vi "Dresden R2R Sputter 03.02.2018 IY24.vi"() -> ()   [LabVIEW 2009] (continued)
                                n28534 = case shown="False" w33549 {
                                frame #0 {
                                n28535 = local read "R Set Pressure mtorr"() -> (w33554:dbl)
                                n28536 = local write "Set_pressure_value 4"(w33554) -> ()
                                }
                                frame #1 {
                                }
                                }
                                }
                                frame #1 {
                                }
                                }
                                }
                                frame #5 {
                                n28537 = local read "Semi"() -> (w33555:bool)
                                n28538 = case shown="False" w33555 {
                                frame #0 {
                                n28539 = local read "Set_pressure_value 4"() -> (w33557:dbl)
                                n28540 = Add(x=1.0, y=w33557) -> (x+y=w33559:dbl)
                                n28541 = Subtract(x=w33557, y=1.0) -> (x-y=w33560:dbl)
                                n28542 = local read "Pressure 4"() -> (w33556:i32)
                                n28543 = In Range and Coerce(upper limit=w33559, x=w33556, lower limit=w33560) -> (In Range?=w33558:bool)  [unwired: 1 out]
                                n28544 = case shown="False" w33558 {
                                frame #0 {
                                n28545 = local write "Pc_bv4_auto_set_pressure"(TRUE ("Pc_bv1_auto_set_pressure")) -> ()
                                }
                                frame #1 {
                                }
                                }
                                }
                                frame #1 {
                                }
                                }
                                }
                                frame #6 {
                                n28546 = local read "Semi"() -> (w33564:bool)
                                n28547 = case shown="False" w33564 {
                                frame #0 {
                                n28548 = while {
                                i -> [w33575]
                                stop <- w33567 stop-if-true
                                n28549 = Greater?(x=w33575, y=300) -> (0:w33569:bool)
                                n28550 = local read "Set_pressure_value 4"() -> (w33566:dbl)
                                n28551 = Add(x=1.0, y=w33566) -> (x+y=w33571:dbl)
                                n28552 = Subtract(x=w33566, y=1.0) -> (x-y=w33572:dbl)
                                n28553 = local read "Pressure 4"() -> (w33565:i32)
                                n28554 = In Range and Coerce(upper limit=w33571, x=w33565, lower limit=w33572) -> (In Range?=w33570:bool)  [unwired: 1 out]
                                n28555 = case shown="False" w33570 {
                                tunnel: [FALSE TRUE] -> w33568
                                frame #0 {
                                n28556 = Wait Until Next ms Multiple(millisecond multiple=u32 200) -> ()  [unwired: 1 out]
                                }
                                frame #1 {
                                }
                                }
                                n28557 = Or(x=w33568, y=w33569) -> (x .or. y?=w33567:bool)
                                }
                                }
                                frame #1 {
                                }
                                }
                                }
                                frame #7 {
                                n28558 = local read "Semi"() -> (w33580:bool)
                                n28559 = case shown="False" w33580 {
                                frame #0 {
                                n28560 = local read "Set_pressure_value 4"() -> (w33582:dbl)
                                n28561 = Add(x=1.0, y=w33582) -> (x+y=w33584:dbl)
                                n28562 = Subtract(x=w33582, y=1.0) -> (x-y=w33585:dbl)
                                n28563 = local read "Pressure 4"() -> (w33581:i32)
                                n28564 = In Range and Coerce(upper limit=w33584, x=w33581, lower limit=w33585) -> (In Range?=w33583:bool)  [unwired: 1 out]
                                n28565 = case shown="False" w33583 {
                                frame #0 {
                                n28566 = local write "Semi"(TRUE ("Semi")) -> ()
                                n28567 = local write "Error Message"("Coating Pressure could not be adjusted !" ("Error Message")) -> ()
                                }
                                frame #1 {
                                }
                                }
                                }
                                frame #1 {
                                }
                                }
                                }
                                }
                                }
                                frame #1 {
                                }
                                }
                                }
                                frame #1 {
                                n28568 = local read "Semi"() -> (w33590:bool)
                                n28569 = case shown="False" w33590 {
                                frame #0 {
                                n28570 = local write "SDC1 9"(TRUE ("SDC1 9")) -> ()
                                n28571 = Wait (ms)(milliseconds to wait=u32 1000) -> ()  [unwired: 1 out]
                                }
                                frame #1 {
                                }
                                }
                                }
                                }
                                }
                                }
                                }
                                frame #15 {
                                # "DC -Ignite Plasma"
                                n28572 = stacked-sequence {
                                frame #0 {
                                n28573 = local read "Semi"() -> (w33593:bool)
                                n28574 = case shown="False" w33593 {
                                frame #0 {
                                n28575 = stacked-sequence {
                                frame #0 {
                                n28576 = local read "Semi"() -> (w33594:bool)
                                n28577 = case shown="False" w33594 {
                                frame #0 {
                                n28578 = local write "RF_host_auto"(TRUE ("Dc_host_auto")) -> ()
                                }
                                frame #1 {
                                }
                                }
                                }
                                frame #1 {
                                n28579 = local read "Semi"() -> (w33596:bool)
                                n28580 = case shown="False" w33596 {
                                frame #0 {
                                n28581 = local read "R Single RF  Step1 Coating Power"() -> (w33597:dbl)
                                n28582 = local write "RF_forward_power_1"(w33597) -> ()
                                }
                                frame #1 {
                                }
                                }
                                }
                                frame #2 {
                                n28583 = local read "Semi"() -> (w33598:bool)
                                n28584 = case shown="False" w33598 {
                                frame #0 {
                                n28585 = Wait (ms)(milliseconds to wait=u32 1000) -> ()  [unwired: 1 out]
                                }
                                frame #1 {
                                }
                                }
                                }
                                frame #3 {
                                n28586 = local read "Semi"() -> (w33600:bool)
                                n28587 = case shown="False" w33600 {
                                frame #0 {
                                n28588 = local write "RF set auto"(TRUE ("Dc_auto_set")) -> ()
                                }
                                frame #1 {
                                }
                                }
                                }
                                frame #4 {
                                n28589 = Wait (ms)(milliseconds to wait=u32 1000) -> ()  [unwired: 1 out]
                                }
                                frame #5 {
                                n28590 = local read "Semi"() -> (w33603:bool)
                                n28591 = case shown="False" w33603 {
                                frame #0 {
                                n28592 = local read "Web_selection_tab"() -> (w33604:T5)
                                n28593 = case shown="\"Other                                                                                    \"" w33604 {
                                frame #0 {
                                }
                                frame #1 {
                                n28594 = local write "RF_auto_on"(TRUE ("Dc_auto_on")) -> ()
                                }
                                }
                                }
                                frame #1 {
                                }
                                }
                                }
                                frame #6 {
                                n28595 = local read "Web_selection_tab"() -> (w33606:T5)
                                n28596 = case shown="\"Other                                                                                    \"" w33606 {
                                frame #0 {
                                }
                                frame #1 {
                                n28597 = local read "Semi"() -> (w33607:bool)
                                n28598 = case shown="False" w33607 {
                                frame #0 {
                                n28599 = while {
                                i -> [w33617]
                                stop <- w33610 stop-if-true
                                n28600 = Greater Or Equal?(x=w33617, y=240) -> (x >= y?=w33616:bool)
                                n28601 = case shown="True" w33616 {
                                frame #0 {
                                }
                                frame #1 {
                                n28602 = local write "Semi"(TRUE ("Semi")) -> ()
                                }
                                }
                                n28603 = local read "RF_forward_power_1"() -> (w33608:i16)
                                n28604 = local read "RF Net Power :"() -> (w33609:u32)
                                n28605 = Subtract(x=w33608, y=w33609) -> (x-y=w33615:u32)
                                n28606 = Less?(x=w33615, y=10.0) -> (x < y?=w33612:bool)
                                n28607 = local read "Semi"() -> (w33611:bool)
                                n28608 = Or(x=w33612, y=w33611) -> (x .or. y?=w33610:bool)
                                n28609 = Wait Until Next ms Multiple(millisecond multiple=u32 500) -> ()  [unwired: 1 out]
                                }
                                }
                                frame #1 {
                                }
                                }
                                }
                                }
                                }
                                frame #7 {
                                n28610 = local read "Semi"() -> (w33620:bool)
                                n28611 = case shown="False" w33620 {
                                frame #0 {
                                n28612 = Wait (ms)(milliseconds to wait=u32 1000) -> ()  [unwired: 1 out]
                                }
                                frame #1 {
                                }
                                }
                                }
                                }
                                }
                                frame #1 {
                                }
                                }
                                }
                                frame #1 {
                                n28613 = local read "Semi"() -> (w33622:bool)
                                n28614 = case shown="False" w33622 {
                                frame #0 {
                                n28615 = Wait (ms)(milliseconds to wait=u32 1000) -> ()  [unwired: 1 out]
                                n28616 = local write "SDC1 13"(TRUE ("SDC1 13")) -> ()
                                }
                                frame #1 {
                                }
                                }
                                }
                                }
                                }
                                frame #16 {
                                n28617 = local read "Web_selection_tab"() -> (w33625:T5)
                                n28618 = case shown="\"Web                                                                                    \", Default" w33625 {
                                frame #0 {
                                n28619 = stacked-sequence {
                                frame #0 {
                                n28620 = local read "R Minimum diameter"() -> (w33626:dbl)
                                n28621 = local read "R Maximum diameter"() -> (w33627:dbl)
                                n28622 = local read "R Web thicness"() -> (w33628:dbl)
                                n28623 = local read "R Web speed(cm/min)"() -> (w33629:dbl)
                                n28624 = Wait (ms)(milliseconds to wait=u32 100) -> ()  [unwired: 1 out]
                                n28625 = local write "Initial Min Diameter"(w33626) -> ()
                                n28626 = local write "Max Diameter"(w33627) -> ()
                                n28627 = local write "Web Thickness"(w33628) -> ()
                                n28628 = local write "Web Speed"(w33629) -> ()
                                }
                                frame #1 {
                                n28629 = local read "R Single RF Step1 Coating Power Active"() -> (w33644:bool)
                                n28630 = local read "R Single RF Step2 Coating Power Active"() -> (w33643:bool)
                                n28631 = local read "R Single RF Step3 Coating Power Active"() -> (w33642:bool)
                                n28632 = local read "R Single RF Step4 Coating Power Active"() -> (w33641:bool)
                                n28633 = local read "R Single RF Step5 Coating Power Active"() -> (w33640:bool)
                                n28634 = Boolean To (0,1)(Boolean=w33644) -> (0, 1=w33639:i16)
                                n28635 = Boolean To (0,1)(Boolean=w33643) -> (0, 1=w33638:i16)
                                n28636 = Boolean To (0,1)(Boolean=w33642) -> (0, 1=w33637:i16)
                                n28637 = Boolean To (0,1)(Boolean=w33641) -> (0, 1=w33636:i16)
                                n28638 = Boolean To (0,1)(Boolean=w33640) -> (0, 1=w33635:i16)
                                n28639 = Compound Arithmetic op=ADD(w33639, w33638, w33637, w33636, w33635) -> (w33633:i16)
                                n28640 = local read "R Single RF Interval length"() -> (w33634:dbl)
                                n28641 = Wait (ms)(milliseconds to wait=u32 200) -> ()  [unwired: 1 out]
                                n28642 = Multiply(x=w33634, y=w33633) -> (x*y=w33632:dbl)
                                n28643 = local write "Total length"(w33632) -> ()
                                }
                                frame #2 {
                                n28644 = local write "Calculate 2"(TRUE ("Calculate_auto")) -> ()
                                n28645 = Wait (ms)(milliseconds to wait=u32 200) -> ()  [unwired: 1 out]
                                }
                                frame #3 {
                                n28646 = local write "Roll_side_select"(enum32{"Left to Right", "Right to Left"}."Left to Right" ("Roll_side_select")) -> ()
                                n28647 = Wait (ms)(milliseconds to wait=u32 200) -> ()  [unwired: 1 out]
                                }
                                frame #4 {
                                n28648 = Wait (ms)(milliseconds to wait=u32 100) -> ()  [unwired: 1 out]
                                n28649 = local write "Parameters_auto_set"(TRUE ("Parameters_auto_set")) -> ()
                                }
                                frame #5 {
                                n28650 = while {
                                i -> [w33655]
                                stop <- w33651 stop-if-true
                                n28651 = Wait Until Next ms Multiple(millisecond multiple=u32 300) -> ()  [unwired: 1 out]
                                n28652 = Greater?(x=w33655, y=100) -> (0:w33652:bool)
                                n28653 = local read "Parameters_auto_set"() -> (w33656:bool)
                                n28654 = case shown="False" w33656 {
                                tunnel: [TRUE FALSE] -> w33653
                                frame #0 {
                                }
                                frame #1 {
                                }
                                }
                                n28655 = Or(x=w33653, y=w33652) -> (x .or. y?=w33651:bool)
                                }
                                }
                                frame #6 {
                                n28656 = local read "R Tension Value"() -> (w33660:dbl)
                                n28657 = Wait (ms)(milliseconds to wait=u32 200) -> ()  [unwired: 1 out]
                                n28658 = local write "TC1_set_value"(w33660) -> ()
                                }
                                frame #7 {
                                n28659 = local write "TC1_auto_set"(TRUE ("TC1_auto_set")) -> ()
                                }
                                frame #8 {
                                w33664 = u16 3 items=["1", "2", "3", "4"] ("Target Chamber Sensor")
                                n28660 = local write "Target Chamber Sensor"(w33664) -> ()
                                n28661 = Wait (ms)(milliseconds to wait=u32 200) -> ()  [unwired: 1 out]
                                }
                                frame #9 {
                                n28662 = local read "Total length"() -> (w33665:dbl)
                                n28663 = local write "Region"(w33665) -> ()
                                }
                                frame #10 {
                                n28664 = local read "Semi"() -> (w33666:bool)
                                n28665 = case shown="False" w33666 {
                                frame #0 {
                                n28666 = stacked-sequence {
                                frame #0 {
                                # "Gas Flow"
                                n28667 = stacked-sequence {
                                frame #0 {
                                n28668 = local read "Semi"() -> (w33667:bool)
                                n28669 = case shown="False" w33667 {
                                frame #0 {
                                n28670 = stacked-sequence {
                                frame #0 {
                                n28671 = local read "Semi"() -> (w33668:bool)
                                n28672 = case shown="False" w33668 {
                                frame #0 {
                                n28673 = local read "R Argon Flow sccm"() -> (w33669:dbl)
                                n28674 = local write "Ar_sccm3_4"(w33669) -> ()
                                }
                                frame #1 {
                                }
                                }
                                }
                                frame #1 {
                                n28675 = local read "Semi"() -> (w33670:bool)
                                n28676 = case shown="False" w33670 {
                                frame #0 {
                                n28677 = local write "Mfc2_Ar _3_4_set"(TRUE ("Mfc_Ar _1_2_set")) -> ()
                                }
                                frame #1 {
                                }
                                }
                                }
                                frame #2 {
                                n28678 = local read "Semi"() -> (w33672:bool)
                                n28679 = case shown="False" w33672 {
                                frame #0 {
                                n28680 = while {
                                i -> [w33675]
                                stop <- w33677 stop-if-true
                                n28681 = Greater?(x=w33675, y=50) -> (0:w33674:bool)
                                n28682 = local read "Semi"() -> (w33673:bool)
                                n28683 = Or(x=w33673, y=w33674) -> (x .or. y?=w33677:bool)
                                }
                                }
                                frame #1 {
                                }
                                }
                                }
                                frame #3 {
                                n28684 = local read "Semi"() -> (w33678:bool)
                                n28685 = case shown="False" w33678 {
                                frame #0 {
                                n28686 = local read "Ar_sccm_act 2"() -> (w33679:dbl)
                                n28687 = Greater?(x=w33679, y=1) -> (0:w33680:bool)
                                n28688 = case shown="False" w33680 {
                                frame #0 {
                                n28689 = local read "R Argon Flow sccm"() -> (w33682:dbl)
                                n28690 = local write "Ar_sccm3_4"(w33682) -> ()
                                }
                                frame #1 {
                                }
                                }
                                }
                                frame #1 {
                                }
                                }
                                }
                                frame #4 {
                                n28691 = local read "Semi"() -> (w33683:bool)
                                n28692 = case shown="False" w33683 {
                                frame #0 {
                                n28693 = local read "Ar_sccm_act 2"() -> (w33684:dbl)
                                n28694 = Greater?(x=w33684, y=1) -> (0:w33685:bool)
                                n28695 = case shown="False" w33685 {
                                frame #0 {
                                n28696 = while {
                                i -> [w33688]
                                stop <- w33692 stop-if-true
                                n28697 = Greater?(x=w33688, y=50) -> (0:w33687:bool)
                                n28698 = local read "Semi"() -> (w33691:bool)
                                n28699 = case shown="False" w33691 {
                                tunnel: [FALSE TRUE] -> w33690
                                frame #0 {
                                n28700 = Wait Until Next ms Multiple(millisecond multiple=u32 200) -> ()  [unwired: 1 out]
                                }
                                frame #1 {
                                }
                                }
                                n28701 = Or(x=w33690, y=w33687) -> (x .or. y?=w33692:bool)
                                }
                                }
                                frame #1 {
                                }
                                }
                                }
                                frame #1 {
                                }
                                }
                                }
                                frame #5 {
                                n28702 = local read "Semi"() -> (w33696:bool)
                                n28703 = case shown="False" w33696 {
                                frame #0 {
                                n28704 = local read "Ar_sccm_act 2"() -> (w33697:dbl)
                                n28705 = Greater?(x=w33697, y=1) -> (0:w33698:bool)
                                n28706 = case shown="False" w33698 {
                                frame #0 {
                                n28707 = local write "Semi"(TRUE ("Semi")) -> ()
                                n28708 = local write "Error Message"("Coating process cancelled.\nPlease check connections." ("Error Message")) -> ()
                                }
                                frame #1 {
                                }
                                }
                                }
                                frame #1 {
                                }
                                }
                                }
                                }
                                }
                                frame #1 {
                                }
                                }
                                }
                                frame #1 {
                                n28709 = local read "Semi"() -> (w33702:bool)
                                n28710 = case shown="False" w33702 {
                                frame #0 {
                                n28711 = local write "SDC1 11"(TRUE ("SDC1 11")) -> ()
                                n28712 = Wait (ms)(milliseconds to wait=u32 1000) -> ()  [unwired: 1 out]
                                }
                                frame #1 {
                                }
                                }
                                }
                                }
                                }
                                frame #1 {
                                # "Set Pressure for ignite plasma"
                                n28713 = stacked-sequence {
                                frame #0 {
                                n28714 = local read "Semi"() -> (w33705:bool)
                                n28715 = case shown="False" w33705 {
                                frame #0 {
                                n28716 = stacked-sequence {
                                frame #0 {
                                n28717 = local read "Semi"() -> (w33706:bool)
                                n28718 = case shown="False" w33706 {
                                frame #0 {
                                n28719 = local write "Set_pressure_value 4"(10.0 ("Set_pressure_value 2")) -> ()
                                }
                                frame #1 {
                                }
                                }
                                }
                                frame #1 {
                                n28720 = local read "Semi"() -> (w33708:bool)
                                n28721 = case shown="False" w33708 {
                                frame #0 {
                                n28722 = Wait (ms)(milliseconds to wait=u32 1000) -> ()  [unwired: 1 out]
                                }
                                frame #1 {
                                }
                                }
                                }
                                frame #2 {
                                n28723 = local read "Semi"() -> (w33710:bool)
                                n28724 = case shown="False" w33710 {
                                frame #0 {
                                n28725 = local write "Pc_bv4_auto_set_pressure"(TRUE ("Pc_bv1_auto_set_pressure")) -> ()
                                }
                                frame #1 {
                                }
                                }
                                }
                                frame #3 {
                                n28726 = local read "Semi"() -> (w33712:bool)
                                n28727 = case shown="False" w33712 {
                                frame #0 {
                                n28728 = while {
                                i -> [w33723]
                                stop <- w33715 stop-if-true
                                w33713 = 10.0 ("Set_pressure_value 2")
                                n28729 = Greater?(x=w33723, y=300) -> (0:w33717:bool)
                                n28730 = Add(x=1.0, y=w33713) -> (x+y=w33719:dbl)
                                n28731 = Subtract(x=w33713, y=1.0) -> (x-y=w33720:dbl)
                                n28732 = local read "Pressure 4"() -> (w33714:i32)
                                n28733 = In Range and Coerce(upper limit=w33719, x=w33714, lower limit=w33720) -> (In Range?=w33718:bool)  [unwired: 1 out]
                                n28734 = case shown="False" w33718 {
                                tunnel: [FALSE TRUE] -> w33716
                                frame #0 {
                                n28735 = Wait Until Next ms Multiple(millisecond multiple=u32 200) -> ()  [unwired: 1 out]
                                }
                                frame #1 {
                                }
                                }
                                n28736 = Or(x=w33716, y=w33717) -> (x .or. y?=w33715:bool)
                                }
                                }
                                frame #1 {
                                }
                                }
                                }
                                frame #4 {
                                n28737 = local read "Semi"() -> (w33728:bool)
                                n28738 = case shown="False" w33728 {
                                frame #0 {
                                w33729 = 10.0 ("Set_pressure_value 2")
                                n28739 = Add(x=1.0, y=w33729) -> (x+y=w33732:dbl)
                                n28740 = Subtract(x=w33729, y=1.0) -> (x-y=w33733:dbl)
                                n28741 = local read "Pressure 4"() -> (w33730:i32)
                                n28742 = In Range and Coerce(upper limit=w33732, x=w33730, lower limit=w33733) -> (In Range?=w33731:bool)  [unwired: 1 out]
                                n28743 = case shown="False" w33731 {
                                frame #0 {
                                n28744 = local read "R Set Pressure mtorr"() -> (w33736:dbl)
                                n28745 = local write "Set_pressure_value 4"(w33736) -> ()
                                }
                                frame #1 {
                                }
                                }
                                }
                                frame #1 {
                                }
                                }
                                }
                                frame #5 {
                                n28746 = local read "Semi"() -> (w33737:bool)
                                n28747 = case shown="False" w33737 {
                                frame #0 {
                                w33738 = 10.0 ("Set_pressure_value 2")
                                n28748 = Add(x=1.0, y=w33738) -> (x+y=w33741:dbl)
                                n28749 = Subtract(x=w33738, y=1.0) -> (x-y=w33742:dbl)
                                n28750 = local read "Pressure 4"() -> (w33739:i32)
                                n28751 = In Range and Coerce(upper limit=w33741, x=w33739, lower limit=w33742) -> (In Range?=w33740:bool)  [unwired: 1 out]
                                n28752 = case shown="False" w33740 {
                                frame #0 {
                                n28753 = local write "Pc_bv4_auto_set_pressure"(TRUE ("Pc_bv1_auto_set_pressure")) -> ()
                                }
                                frame #1 {
                                }
                                }
                                }
                                frame #1 {
                                }
                                }
                                }
                                frame #6 {
                                n28754 = local read "Semi"() -> (w33746:bool)
                                n28755 = case shown="False" w33746 {
                                frame #0 {
                                n28756 = while {
                                i -> [w33757]
                                stop <- w33749 stop-if-true
                                w33747 = 10.0 ("Set_pressure_value 2")
                                n28757 = Greater?(x=w33757, y=300) -> (0:w33751:bool)
                                n28758 = Add(x=1.0, y=w33747) -> (x+y=w33753:dbl)
                                n28759 = Subtract(x=w33747, y=1.0) -> (x-y=w33754:dbl)
                                n28760 = local read "Pressure 4"() -> (w33748:i32)
                                n28761 = In Range and Coerce(upper limit=w33753, x=w33748, lower limit=w33754) -> (In Range?=w33752:bool)  [unwired: 1 out]
                                n28762 = case shown="False" w33752 {
                                tunnel: [FALSE TRUE] -> w33750
                                frame #0 {
                                n28763 = Wait Until Next ms Multiple(millisecond multiple=u32 200) -> ()  [unwired: 1 out]
                                }
                                frame #1 {
                                }
                                }
                                n28764 = Or(x=w33750, y=w33751) -> (x .or. y?=w33749:bool)
                                }
                                }
                                frame #1 {
                                }
                                }
                                }
                                frame #7 {
                                n28765 = local read "Semi"() -> (w33762:bool)
                                n28766 = case shown="False" w33762 {
                                frame #0 {
                                n28767 = local read "Set_pressure_value 4"() -> (w33765:dbl)
                                n28768 = Add(x=1.0, y=w33765) -> (x+y=w33766:dbl)
                                n28769 = Subtract(x=w33765, y=1.0) -> (x-y=w33767:dbl)
                                n28770 = local read "Pressure 4"() -> (w33763:i32)
                                n28771 = In Range and Coerce(upper limit=w33766, x=w33763, lower limit=w33767) -> (In Range?=w33764:bool)  [unwired: 1 out]
                                n28772 = case shown="False" w33764 {
                                frame #0 {
                                n28773 = local write "Semi"(TRUE ("Semi")) -> ()
                                n28774 = local write "Error Message"("Coating Pressure could not be adjusted !" ("Error Message")) -> ()
                                }
                                frame #1 {
                                }
                                }
                                }
                                frame #1 {
                                }
                                }
                                }
                                }
                                }
                                frame #1 {
                                }
                                }
                                }
                                frame #1 {
                                n28775 = local read "Semi"() -> (w33772:bool)
                                n28776 = case shown="False" w33772 {
                                frame #0 {
                                n28777 = local write "SDC1 9"(TRUE ("SDC1 9")) -> ()
                                n28778 = Wait (ms)(milliseconds to wait=u32 1000) -> ()  [unwired: 1 out]
                                }
                                frame #1 {
                                }
                                }
                                }
                                }
                                }
                                frame #2 {
                                # "Plasma ignite and check"
                                n28779 = stacked-sequence {
                                frame #0 {
                                n28780 = local read "Semi"() -> (w33775:bool)
                                n28781 = case shown="False" w33775 {
                                frame #0 {
                                n28782 = local write "RF_auto_on"(TRUE ("Dc_auto_on")) -> ()
                                }
                                frame #1 {
                                }
                                }
                                }
                                frame #1 {
                                n28783 = local read "Semi"() -> (w33777:bool)
                                n28784 = case shown="False" w33777 {
                                frame #0 {
                                n28785 = while {
                                i -> [w33787]
                                stop <- w33779 stop-if-true
                                n28786 = Greater Or Equal?(x=w33787, y=240) -> (x >= y?=w33786:bool)
                                n28787 = case shown="True" w33786 {
                                frame #0 {
                                }
                                frame #1 {
                                n28788 = local write "Semi"(TRUE ("Semi")) -> ()
                                }
                                }
                                n28789 = local read "RF Net Power :"() -> (w33778:u32)
                                n28790 = local read "RF_forward_power_1"() -> (w33783:i16)
                                n28791 = Subtract(x=w33783, y=w33778) -> (x-y=w33785:u32)
                                n28792 = Less?(x=w33785, y=10.0) -> (x < y?=w33781:bool)
                                n28793 = local read "Semi"() -> (w33780:bool)
                                n28794 = Or(x=w33781, y=w33780) -> (x .or. y?=w33779:bool)
                                n28795 = Wait Until Next ms Multiple(millisecond multiple=u32 500) -> ()  [unwired: 1 out]
                                }
                                }
                                frame #1 {
                                }
                                }
                                }
                                }
                                }
                                frame #3 {
                                # "Set Pressure for coating"
                                n28796 = stacked-sequence {
                                frame #0 {
                                n28797 = local read "Semi"() -> (w33790:bool)
                                n28798 = case shown="False" w33790 {
                                frame #0 {
                                n28799 = stacked-sequence {
                                frame #0 {
                                n28800 = local read "Semi"() -> (w33791:bool)
                                n28801 = case shown="False" w33791 {
                                frame #0 {
                                n28802 = local read "R Set Pressure mtorr"() -> (w33792:dbl)
                                n28803 = local write "Set_pressure_value 4"(w33792) -> ()
                                }
                                frame #1 {
                                }
                                }
                                }
                                frame #1 {
                                n28804 = local read "Semi"() -> (w33793:bool)
                                n28805 = case shown="False" w33793 {
                                frame #0 {
                                n28806 = Wait (ms)(milliseconds to wait=u32 200) -> ()  [unwired: 1 out]
                                }
                                frame #1 {
                                }
                                }
                                }
                                frame #2 {
                                n28807 = local read "Semi"() -> (w33795:bool)
                                n28808 = case shown="False" w33795 {
                                frame #0 {
                                n28809 = local write "Pc_bv4_auto_set_pressure"(TRUE ("Pc_bv1_auto_set_pressure")) -> ()
                                }
                                frame #1 {
                                }
                                }
                                }
                                frame #3 {
                                n28810 = local read "Semi"() -> (w33797:bool)
                                n28811 = case shown="False" w33797 {
                                frame #0 {
                                n28812 = while {
                                i -> [w33808]
                                stop <- w33800 stop-if-true
                                n28813 = local read "Set_pressure_value 4"() -> (w33798:dbl)
                                n28814 = Greater?(x=w33808, y=300) -> (0:w33802:bool)
                                n28815 = Add(x=1.0, y=w33798) -> (x+y=w33804:dbl)
                                n28816 = Subtract(x=w33798, y=1.0) -> (x-y=w33805:dbl)
                                n28817 = local read "Pressure 4"() -> (w33799:i32)
                                n28818 = In Range and Coerce(upper limit=w33804, x=w33799, lower limit=w33805) -> (In Range?=w33803:bool)  [unwired: 1 out]
                                n28819 = case shown="False" w33803 {
                                tunnel: [FALSE TRUE] -> w33801
                                frame #0 {
                                n28820 = Wait Until Next ms Multiple(millisecond multiple=u32 200) -> ()  [unwired: 1 out]
                                }
                                frame #1 {
                                }
                                }
                                n28821 = Or(x=w33801, y=w33802) -> (x .or. y?=w33800:bool)
                                }
                                }
                                frame #1 {
                                }
                                }
                                }
                                frame #4 {
                                n28822 = local read "Semi"() -> (w33813:bool)
                                n28823 = case shown="False" w33813 {
                                frame #0 {
                                n28824 = local read "Set_pressure_value 4"() -> (w33814:dbl)
                                n28825 = Add(x=1.0, y=w33814) -> (x+y=w33817:dbl)
                                n28826 = Subtract(x=w33814, y=1.0) -> (x-y=w33818:dbl)
                                n28827 = local read "Pressure 4"() -> (w33815:i32)
                                n28828 = In Range and Coerce(upper limit=w33817, x=w33815, lower limit=w33818) -> (In Range?=w33816:bool)  [unwired: 1 out]
                                n28829 = case shown="False" w33816 {
                                frame #0 {
                                n28830 = local read "R Set Pressure mtorr"() -> (w33821:dbl)
                                n28831 = local write "Set_pressure_value 4"(w33821) -> ()
                                }
                                frame #1 {
                                }
                                }
                                }
                                frame #1 {
                                }
                                }
                                }
                                frame #5 {
                                n28832 = local read "Semi"() -> (w33822:bool)
                                n28833 = case shown="False" w33822 {
                                frame #0 {
                                n28834 = local read "Set_pressure_value 4"() -> (w33823:dbl)
                                n28835 = Add(x=1.0, y=w33823) -> (x+y=w33826:dbl)
                                n28836 = Subtract(x=w33823, y=1.0) -> (x-y=w33827:dbl)
                                n28837 = local read "Pressure 4"() -> (w33824:i32)
                                n28838 = In Range and Coerce(upper limit=w33826, x=w33824, lower limit=w33827) -> (In Range?=w33825:bool)  [unwired: 1 out]